vi "HFRR ADV v037.vi"() -> ()   [LabVIEW 2025] (continued)
                            n2633 = local write "Batch Ref Num :"(w3119) -> ()
                            n2634 = local write "FILE"(w3119) -> ()
                            n2635 = local write "EVENT LOG"(w3124) -> ()
                            n2636 = local write "TEST FILE NAM,E SAVED"(w3117) -> ()
                            n2637 = local write "Fuel Discription :"(w3119) -> ()
                            n2638 = local write "START TEMP"(w3117) -> ()
                            n2639 = local write "Remarks :"(w3119) -> ()
                            n2640 = local write "Main Dashboard Buttons"(T1."Imaging" ("Main Dashboard Buttons")) -> ()
                            n2641 = local write "Main Tab"(T2."Adv Scar" ("Main Tab")) -> ()
                            n2642 = property on="FRICVALZ 2" class="Bool (strict)"("DisabledEnum"=w3118) -> ()  [unwired: 2 in, 2 out]
                            n2643 = property on="FRICVALZ 3" class="Bool (strict)"("DisabledEnum"=w3118) -> ()  [unwired: 2 in, 2 out]
                            n2644 = property on="FRICVALZ 4" class="Bool (strict)"("DisabledEnum"=w3118) -> ()  [unwired: 2 in, 2 out]
                          }
                          frame #1 {
                            n2645 = Wait (ms)(milliseconds to wait=u32 1500) -> ()  [unwired: 1 out]
                          }
                          frame #2 {
                            n2646 = local write "Due Write"("VC;0") -> ()
                          }
                          frame #3 {
                            n2647 = Wait (ms)(milliseconds to wait=u32 1500) -> ()  [unwired: 1 out]
                          }
                          frame #4 {
                            n2648 = local write "Due Write"("VC;0") -> ()
                          }
                          frame #5 {
                            n2649 = Wait (ms)(milliseconds to wait=u32 1500) -> ()  [unwired: 1 out]
                          }
                          frame #6 {
                            n2650 = local write "Due Write"("ST;0") -> ()
                          }
                          frame #7 {
                            n2651 = local write "measured_stroke"(0.0 ("measured_stroke")) -> ()
                            n2652 = Wait (ms)(milliseconds to wait=u32 1500) -> ()  [unwired: 1 out]
                          }
                          frame #8 {
                            n2653 = local write "Due Write"("HE;0") -> ()
                            n2654 = local write "Humidity"(TRUE ("Humidity")) -> ()
                          }
                        }
                      }
                    }
                    n2655 = Divide(x=w3102, y=w3101) -> (x/y=w3105:dbl)
                    n2656 = Multiply(x=w3105, y=100.0) -> (x*y=w3103:dbl)
                    n2657 = local write "Test Duration Status"(w3103) -> ()
                  }
                }
              }
              frame #2 {
                n2658 = case shown="True" "Heater Button" {
                  tunnel: [0.0 ("output") w3240] -> w3218
                  frame False {
                    w3221 = TRUE ("tmpchk")
                    n2659 = local read "TEMP"() -> (w3222:dbl)
                    n2660 = local write "Temp ini"(w3222) -> ()
                    n2661 = local write "Reset 4"(w3221) -> ()
                    n2662 = local write "tmpchk"(w3221) -> ()
                    n2663 = local write "reinit"(TRUE ("reinit")) -> ()
                    n2664 = local write "manual temp log"(TRUE ("manual temp log")) -> ()
                  }
                  frame True {
                    # "Logic to turn off\nthe heater when \ntemp is not rising.\nTime - 60 sec\nDelta t- 5°c"
                    n2665 = local read "Temp ini"() -> (w3229:dbl)
                    n2666 = local read "Auto Start Test"() -> (w3225:bool)
                    n2667 = Less?(x=w3229, y=53.0) -> (x < y?=w3227:bool)
                    n2668 = case shown="False" w3225 {
                      frame False {
                        n2669 = local read "Set Temp"() -> (w3249:dbl)
                        n2670 = local read "TEMP"() -> (w3248:dbl)
                        n2671 = Subtract(x=w3249, y=w3248) -> (x-y=w3247:dbl)
                        n2672 = Absolute Value(x=w3247) -> (abs(x)=w3246:dbl)
                        n2673 = Less?(x=w3246, y=0.5) -> (x < y?=w3244:bool)
                        n2674 = case shown="True" w3244 {
                          tunnel: "manual temp log" -> [_ w3250]
                          frame False {
                          }
                          frame True {
                            n2675 = case shown="True" w3250 {
                              selector: w3250 -> [_ w3251]
                              frame False {
                              }
                              frame True {
                                # "#Event log"
                                n2676 = Not(x=w3251) -> (.not. x?=w3252:bool)
                                n2677 = local write "manual temp log"(w3252) -> ()
                                n2678 = local read "EVENT LOG"() -> (w3255:string)
                                n2679 = call "Event Log.vi"("Content"="Target Temperature reached", "EVENT LOG"=w3255) -> ("EVENT LOG"=w3254:string)  [unwired: 8 in, 1 out]
                                n2680 = local write "EVENT LOG"(w3254) -> ()
                              }
                            }
                          }
                        }
                      }
                      frame True {
                        n2681 = local write "manual temp log"(TRUE ("manual temp log")) -> ()
                      }
                    }
                    n2682 = And(x="tmpchk", y=w3227) -> (x .and. y?=w3230:bool)
                    n2683 = case shown="True" w3230 {
                      frame False {
                      }
                      frame True {
                        n2684 = call "Elapsed Time8"("Time Target (s)"=300.0, "Reset"="Reset 4") -> ("Time has Elapsed"=w3257:bool)  [unwired: 10 in, 7 out]
                        n2685 = flat-sequence {
                          tunnel: w3257 -> [_]
                          frame #0 {
                            n2686 = local write "Reset 4"(FALSE ("Reset 4")) -> ()
                          }
                        }
                        n2687 = case shown="True" w3257 {
                          frame False {
                          }
                          frame True {
                            n2688 = local read "Temp ini"() -> (w3264:dbl)
                            n2689 = Add(x=w3264, y=5.0) -> (x+y=w3262:dbl)
                            n2690 = local read "TEMP"() -> (w3265:dbl)
                            n2691 = Greater?(x=w3265, y=w3262) -> (0:w3263:bool)
                            n2692 = case shown="False" w3263 {
                              frame False {
                                n2693 = local write "Heater Button"(FALSE ("Heater Button")) -> ()
                              }
                              frame True {
                                n2694 = local write "tmpchk"(FALSE ("tmpchk")) -> ()
                              }
                            }
                          }
                        }
                      }
                    }
                    n2695 = local read "Set Temp"() -> (w3238:dbl)
                    n2696 = local read "TEMP"() -> (w3232:dbl)
                    n2697 = call-poly <vilib>:"PID.vi"("reinitialize? (F)"="reinit", "dt (s)"=-1.0, "process variable"=w3232, "setpoint"=w3238) -> ("output"=w3235:dbl)  [unwired: 6 in, 1 out]
                    n2698 = Subtract(x=w3238, y=w3232) -> (x-y=w3239:dbl)
                    n2699 = Add(x=w3238, y=0.5) -> (x+y=w3236:dbl)
                    n2700 = Greater Or Equal?(x=w3232, y=w3236) -> ()  [unwired: 1 out]
                    n2701 = Select(t=0.0, s=FALSE, f=w3235) -> (s? t:f=w3234:dbl)
                    "PID output" <- w3234
                    n2702 = flat-sequence {
                      tunnel: w3234 -> [w3268]
                      tunnel: [w3268] -> w3240
                      frame #0 {
                        n2703 = local write "reinit"(FALSE ("reinit")) -> ()
                      }
                    }
                    n2704 = Bundle(w3239, "output"=w3234, "TEMP"=w3232) -> ()  [unwired: 1 in, 1 out]
                  }
                }
                "PID-out" <- w3218
              }
              frame #3 {
                n2705 = local read "TEMP"() -> (w3270:dbl)
                n2706 = Greater Or Equal?(x=w3270, y="Set Temp 2") -> (x >= y?=w3275:bool)
                n2707 = case shown="True" w3275 {
                  tunnel: [FALSE TRUE] -> w3273
                  frame False {
                  }
                  frame True {
                  }
                }
                "Status 13" <- w3273
                n2708 = And(x=w3273, y="trip1 8") -> (x .and. y?=w3272:bool)
                n2709 = case shown="True" w3272 {
                  frame False {
                    n2710 = local write "Heater Trip Temp"(TRUE ("Heater Trip Temp")) -> ()
                  }
                  frame True {
                    w3278 = FALSE ("OK Button 2")
                    n2711 = case shown="True" "Heater Trip Temp" {
                      selector: "Heater Trip Temp" -> [_ w3280]
                      frame False {
                      }
                      frame True {
                        n2712 = Not(x=w3280) -> (.not. x?=w3279:bool)
                        n2713 = local read "EVENT LOG"() -> (w3283:string)
                        n2714 = local write "Heater Trip Temp"(w3279) -> ()
                        n2715 = call "Event Log.vi"("Content"="Heater Trip", "EVENT LOG"=w3283) -> ("EVENT LOG"=w3282:string)  [unwired: 8 in, 1 out]
                        n2716 = local write "EVENT LOG"(w3282) -> ()
                      }
                    }
                    n2717 = local write "RUN"(w3278) -> ()
                    n2718 = property on="Auto Start Test" class="Bool (strict)"("Value"=w3278) -> ()  [unwired: 2 in, 2 out]
                    n2719 = local write "Heater Button"(w3278) -> ()
                  }
                }
              }
            }
            n2720 = case shown="False" w2989 {
              frame False {
                n2721 = disable-structure shown="Disabled" {
                  frame Disabled {
                    n2722 = stacked-sequence {
                      frame #0 {
                        n2723 = local write "RUN"(FALSE ("OK Button 2")) -> ()
                      }
                      frame #1 {
                      }
                    }
                  }
                  frame Enabled {
                  }
                }
              }
              frame True {
              }
            }
          }
        }
        n2724 = local read "Reset Graph"() -> (w2886:bool)
        n2725 = case shown="True" w2886 {
          selector: w2886 -> [_ w2903]
          frame False {
          }
          frame True {
            w2917 = 0.0 ("X Scale.Range:Maximum")
            n2726 = Not(x=w2903) -> (.not. x?=w2902:bool)
            n2727 = local write "Reset Graph"(w2902) -> ()
            n2728 = property on="Electrical Contact Resistance ( % )" class="WFChart (strict)"("XScale.Maximum"=600.0 ("X Scale.Range:Maximum"), "XScale.Minimum"=0.0 ("X Scale.Range:Minimum"), "YScale.Maximum"=100.0 ("Y Scale.Range:Maximum"), "YScale.Minimum"=0.0 ("Y Scale.Range:Minimum")) -> ()  [unwired: 2 in, 2 out]
            n2729 = property on="Frictional Force ( N )" class="WFChart (strict)"("XScale.Maximum"=600.0 ("X Scale.Range:Maximum"), "XScale.Minimum"=0.0 ("X Scale.Range:Minimum"), "YScale.Maximum"=100.0 ("Y Scale.Range:Maximum"), "YScale.Minimum"=0.0 ("Y Scale.Range:Minimum")) -> ()  [unwired: 2 in, 2 out]
            n2730 = property on="Temperature ( Deg C )" class="WFChart (strict)"("XScale.Maximum"=600.0 ("X Scale.Range:Maximum"), "XScale.Minimum"=0.0 ("X Scale.Range:Minimum"), "YScale.Maximum"=100.0 ("Y Scale.Range:Maximum"), "YScale.Minimum"=0.0 ("Y Scale.Range:Minimum")) -> ()  [unwired: 2 in, 2 out]
            n2731 = property on="Stroke ( mm )" class="WFChart (strict)"("XScale.Maximum"=600.0 ("X Scale.Range:Maximum"), "XScale.Minimum"=0.0 ("X Scale.Range:Minimum"), "YScale.Maximum"=100.0 ("Y Scale.Range:Maximum"), "YScale.Minimum"=0.0 ("Y Scale.Range:Minimum")) -> ()  [unwired: 2 in, 2 out]
            n2732 = property on="Coefficient of Friction" class="WFChart (strict)"("XScale.Maximum"=600.0 ("X Scale.Range:Maximum"), "XScale.Minimum"=0.0 ("X Scale.Range:Minimum"), "YScale.Maximum"=100.0 ("Y Scale.Range:Maximum"), "YScale.Minimum"=0.0 ("Y Scale.Range:Minimum")) -> ()  [unwired: 2 in, 2 out]
            n2733 = property on="Electrical Contact Resistance ( % )" class="WFChart (strict)"("XScale.Minimum"=0.0 ("X Scale.Range:Minimum"), "XScale.Maximum"=600.0 ("X Scale.Range:Maximum"), "YScale.Minimum"=0.0 ("Y Scale.Range:Minimum"), "YScale.Maximum"=100.0 ("Y Scale.Range:Maximum")) -> ()  [unwired: 2 in, 2 out]
            n2734 = property on="Temperature ( Deg C )" class="WFChart (strict)"("XScale.Minimum"=0.0 ("X Scale.Range:Minimum"), "XScale.Maximum"=600.0 ("X Scale.Range:Maximum"), "YScale.Minimum"=0.0 ("Y Scale.Range:Minimum"), "YScale.Maximum"=100.0 ("Y Scale.Range:Maximum")) -> ()  [unwired: 2 in, 2 out]
            n2735 = property on="Coefficient of Friction" class="WFChart (strict)"("XScale.Minimum"=0.0 ("X Scale.Range:Minimum"), "XScale.Maximum"=600.0 ("X Scale.Range:Maximum"), "YScale.Maximum"=1.0 ("X Scale.Range:Minimum"), "YScale.Minimum"=0.0 ("X Scale.Range:Minimum")) -> ()  [unwired: 2 in, 2 out]
            n2736 = property on="Frictional Force ( N )" class="WFChart (strict)"("XScale.Maximum"=600.0 ("X Scale.Range:Maximum"), "XScale.Minimum"=w2917, "YScale.Maximum"=10.0 ("Y Scale.Range:Maximum"), "YScale.Minimum"=w2917) -> ()  [unwired: 2 in, 2 out]
            n2737 = property on="Stroke ( mm )" class="WFChart (strict)"("XScale.Maximum"=600.0 ("X Scale.Range:Maximum"), "XScale.Minimum"=0.0 ("X Scale.Range:Minimum"), "YScale.Maximum"=100.0 ("Y Scale.Range:Maximum"), "YScale.Minimum"=0.0 ("Y Scale.Range:Minimum")) -> ()  [unwired: 2 in, 2 out]
          }
        }
      }
      frame "Compare Files" {
        # "Elapsed time\ncof\nstroke\nAir temp\nTemp\nHumidity"
        n2738 = case shown="True" "RSTV1 2" {
          frame False {
          }
          frame True {
            n2739 = property on="Humidity ( %RH )" class="XYGraph (strict)"("Y Scale.Display Format:Precision"=u8 0 ("Y Scale.Format & Precision:Precision")) -> ()  [unwired: 2 in, 2 out]
            n2740 = property on="Humidity ( %RH )" class="XYGraph (strict)"("X Scale.Range:Minimum"=0.0, "X Scale.Range:Maximum"=75.0, "Y Scale.Range:Minimum"=48.0, "Y Scale.Range:Maximum"=58.0) -> ()  [unwired: 2 in, 2 out]
          }
        }
        n2741 = case shown="True" "RST CP 2" {
          frame False {
          }
          frame True {
            n2742 = property on="XY Graph 13" class="XYGraph (strict)"("Y Scale.Display Format:Precision"=u8 0 ("Y Scale.Format & Precision:Precision")) -> ()  [unwired: 2 in, 2 out]
            n2743 = property on="XY Graph 13" class="XYGraph (strict)"("X Scale.Range:Minimum"=0.0, "X Scale.Range:Maximum"=75.0, "Y Scale.Range:Minimum"=0.0, "Y Scale.Range:Maximum"=100.0) -> ()  [unwired: 2 in, 2 out]
          }
        }
        n2744 = case shown="True" "RST CP" {
          frame False {
          }
          frame True {
            n2745 = property on="Sample Temperature ( °C )" class="XYGraph (strict)"("Y Scale.Display Format:Precision"=u8 2 ("Y Scale.Format & Precision:Precision")) -> ()  [unwired: 2 in, 2 out]
            n2746 = property on="Sample Temperature ( °C )" class="XYGraph (strict)"("X Scale.Range:Minimum"=0.0, "X Scale.Range:Maximum"=75.0, "Y Scale.Range:Minimum"=58.0, "Y Scale.Range:Maximum"=62.0) -> ()  [unwired: 2 in, 2 out]
          }
        }
        n2747 = case shown="True" "RSTV1 3" {
          frame False {
          }
          frame True {
            n2748 = property on="Air Temperature  ( °C )" class="XYGraph (strict)"("Y Scale.Display Format:Precision"=u8 2 ("Y Scale.Format & Precision:Precision")) -> ()  [unwired: 2 in, 2 out]
            n2749 = property on="Air Temperature  ( °C )" class="XYGraph (strict)"("X Scale.Range:Minimum"=0.0 ("Y Scale.Range:Minimum"), "X Scale.Range:Maximum"=75.0 ("Y Scale.Range:Maximum"), "Y Scale.Range:Minimum"=20.0 ("X Scale.Range:Minimum"), "Y Scale.Range:Maximum"=26.0 ("X Scale.Range:Maximum")) -> ()  [unwired: 2 in, 2 out]
          }
        }
        n2750 = case shown="True" "RSTV1 4" {
          frame False {
          }
          frame True {
            n2751 = property on="Stroke ( mm )" class="XYGraph (strict)"("Y Scale.Display Format:Precision"=u8 2 ("Y Scale.Format & Precision:Precision")) -> ()  [unwired: 2 in, 2 out]
            n2752 = property on="Stroke ( mm )" class="XYGraph (strict)"("X Scale.Range:Minimum"=0.0 ("Y Scale.Range:Maximum"), "X Scale.Range:Maximum"=75.0 ("X Scale.Range:Minimum"), "Y Scale.Range:Minimum"=0.98, "Y Scale.Range:Maximum"=1.02) -> ()  [unwired: 2 in, 2 out]
          }
        }
        n2753 = case shown="True" "rstv2" {
          frame False {
          }
          frame True {
            n2754 = property on="Coefficient Of Friction" class="XYGraph (strict)"("Y Scale.Display Format:Precision"=u8 3 ("Y Scale.Format & Precision:Precision")) -> ()  [unwired: 2 in, 2 out]
            n2755 = property on="Coefficient Of Friction" class="XYGraph (strict)"("X Scale.Range:Minimum"=0.0 ("Y Scale.Range:Maximum"), "X Scale.Range:Maximum"=75.0, "Y Scale.Range:Minimum"=0.0, "Y Scale.Range:Maximum"=1.0 ("X Scale.Range:Minimum")) -> ()  [unwired: 2 in, 2 out]
          }
        }
        n2756 = case shown="True" "RST CP 3" {
          frame False {
          }
          frame True {
            n2757 = property on="Air Temp ( °C ) vs Humidity ( % RH )" class="XYGraph (strict)"("X Scale.Range:Minimum"=18.0, "X Scale.Range:Maximum"=28.0 ("X Scale.Range:Minimum"), "Y Scale.Range:Minimum"=30.0 ("X Scale.Range:Minimum"), "Y Scale.Range:Maximum"=70.0 ("X Scale.Range:Minimum")) -> ()  [unwired: 2 in, 2 out]
          }
        }
        n2758 = case shown="True" "OPEN 1" {
          frame False {
          }
          frame True {
            (unwired) 0  # existing file
            w3559 = "Choose a datalog file to open"  # prompt
            n2759 = local write "OPEN 1"(FALSE ("OPEN 1")) -> ()
            n2760 = String To Path(string="C:\\LAB-IQ\\Data\\") -> (path=w3544:path)
            n2761 = File Dialog(6:"*.dgf" ("pattern"), 7:w3559, 11:w3544) -> (0:w3542:errorcluster, 3:w3550:path)  [unwired: 4 in, 2 out]
            n2762 = Unbundle(w3542) -> ()  [unwired: 3 out]
            n2763 = Strip Path(path=w3550) -> (name=w3549:string)  [unwired: 1 out]
            n2764 = Path To String(path=w3550) -> (string=w3545:string)
            "string1" <- w3545
            n2765 = Match Pattern(string=w3549, regular expression=".dgf") -> (before substring=→"String Control":string)  [unwired: 1 in, 3 out]
            n2766 = Match Pattern(string=w3545, regular expression=".dgf" ("substring (\"\")")) -> (before substring=w3555:string)  [unwired: 1 in, 3 out]
            n2767 = Concatenate Strings(w3555, ".duf" ("Substring")) -> (w3551:string)
            n2768 = String To Path(string=w3551) -> (path=w3556:path)
            n2769 = call <vilib>:"Read Characters From File.vi"("file path (dialog if empty)"=w3556, "start of read offset (chars.:0)"=60 ("start of read offset (chars.: 0)")) -> ("character string"=→"String Control 2":string)  [unwired: 4 in, 3 out]
          }
        }
        n2770 = case shown="True" "OPEN 2" {
          frame False {
          }
          frame True {
            (unwired) 0  # existing file
            w3577 = "Choose a datalog file to open"  # prompt
            n2771 = local write "OPEN 2"(FALSE ("OPEN 1")) -> ()
            n2772 = String To Path(string="C:\\LAB-IQ\\Data\\") -> (path=w3562:path)
            n2773 = File Dialog(6:"*.dgf" ("pattern"), 7:w3577, 11:w3562) -> (0:w3560:errorcluster, 3:w3568:path)  [unwired: 4 in, 2 out]
            n2774 = Unbundle(w3560) -> ()  [unwired: 3 out]
            n2775 = Strip Path(path=w3568) -> (name=w3566:string)  [unwired: 1 out]
            n2776 = Path To String(path=w3568) -> (string=w3563:string)
            "string1 2" <- w3563
            n2777 = Match Pattern(string=w3566, regular expression=".dgf") -> (before substring=→"String Control 3":string)  [unwired: 1 in, 3 out]
            n2778 = Match Pattern(string=w3563, regular expression=".dgf" ("substring (\"\")")) -> (before substring=w3574:string)  [unwired: 1 in, 3 out]
            n2779 = Concatenate Strings(w3574, ".duf" ("Substring")) -> (w3571:string)
            n2780 = String To Path(string=w3571) -> (path=w3569:path)
            n2781 = call <vilib>:"Read Characters From File.vi"("file path (dialog if empty)"=w3569, "start of read offset (chars.:0)"=60 ("start of read offset (chars.: 0)")) -> ("character string"=→"String Control 4":string)  [unwired: 4 in, 3 out]
          }
        }
        n2782 = case shown="True" "OPEN 3" {
          frame False {
          }
          frame True {
            (unwired) 0  # existing file
            w3595 = "Choose a datalog file to open"  # prompt
            n2783 = local write "OPEN 3"(FALSE ("OPEN 1")) -> ()
            n2784 = String To Path(string="C:\\LAB-IQ\\Data\\") -> (path=w3580:path)
            n2785 = File Dialog(6:"*.dgf" ("pattern"), 7:w3595, 11:w3580) -> (0:w3578:errorcluster, 3:w3586:path)  [unwired: 4 in, 2 out]
            n2786 = Unbundle(w3578) -> ()  [unwired: 3 out]
            n2787 = Strip Path(path=w3586) -> (name=w3584:string)  [unwired: 1 out]
            n2788 = Path To String(path=w3586) -> (string=w3581:string)
            "string1 3" <- w3581
            n2789 = Match Pattern(string=w3584, regular expression=".dgf") -> (before substring=→"String Control 5":string)  [unwired: 1 in, 3 out]
            n2790 = Match Pattern(string=w3581, regular expression=".dgf" ("substring (\"\")")) -> (before substring=w3591:string)  [unwired: 1 in, 3 out]
            n2791 = Concatenate Strings(w3591, ".duf" ("Substring")) -> (w3588:string)
            n2792 = String To Path(string=w3588) -> (path=w3592:path)
            n2793 = call <vilib>:"Read Characters From File.vi"("file path (dialog if empty)"=w3592, "start of read offset (chars.:0)"=60 ("start of read offset (chars.: 0)")) -> ("character string"=→"String Control 6":string)  [unwired: 4 in, 3 out]
          }
        }
        n2794 = case shown="True" "OPEN 4" {
          frame False {
          }
          frame True {
            (unwired) 0  # existing file
            w3613 = "Choose a datalog file to open"  # prompt
            n2795 = local write "OPEN 4"(FALSE ("OPEN 1")) -> ()
            n2796 = String To Path(string="C:\\LAB-IQ\\Data\\") -> (path=w3598:path)
            n2797 = File Dialog(6:"*.dgf" ("pattern"), 7:w3613, 11:w3598) -> (0:w3596:errorcluster, 3:w3604:path)  [unwired: 4 in, 2 out]
            n2798 = Unbundle(w3596) -> ()  [unwired: 3 out]
            n2799 = Strip Path(path=w3604) -> (name=w3602:string)  [unwired: 1 out]
            n2800 = Path To String(path=w3604) -> (string=w3599:string)
            "string1 4" <- w3599
            n2801 = Match Pattern(string=w3602, regular expression=".dgf") -> (before substring=→"String Control 7":string)  [unwired: 1 in, 3 out]
            n2802 = Match Pattern(string=w3599, regular expression=".dgf" ("substring (\"\")")) -> (before substring=w3609:string)  [unwired: 1 in, 3 out]
            n2803 = Concatenate Strings(w3609, ".duf" ("Substring")) -> (w3606:string)
            n2804 = String To Path(string=w3606) -> (path=w3610:path)
            n2805 = call <vilib>:"Read Characters From File.vi"("file path (dialog if empty)"=w3610, "start of read offset (chars.:0)"=60 ("start of read offset (chars.: 0)")) -> ("character string"=→"String Control 8":string)  [unwired: 4 in, 3 out]
          }
        }
      }
      frame "About" {
        # "Elapsed time\ncof\nstroke\nmean pos\nTemp\nHumidity"
        n2806 = disable-structure shown="Disabled" {
          frame Disabled {
            n2807 = case shown="True" "Export" {
              frame False {
              }
              frame True {
                w3635 = "                                      " ("string")
                w3637 = "\r"
                (unwired) i16 6 ("width (-)")
                w3714 = "\r"
                w3646 = "\r"
                n2808 = local write "Export"(FALSE ("Export")) -> ()
                n2809 = local read "String 29"() -> (w3683:string)
                n2810 = local read "String 34"() -> (w3671:string)
                n2811 = local read "String 35"() -> (w3666:string)
                n2812 = local read "String 37"() -> (w3662:string)
                n2813 = local read "String 36"() -> (w3659:string)
                n2814 = local read "String 38"() -> (w3656:string)
                n2815 = local read "String 39"() -> (w3653:string)
                n2816 = Match Pattern(string=w3683, regular expression=".dwm") -> (before substring=w3679:string)  [unwired: 1 in, 3 out]
                "before substring" <- w3679
                n2817 = local read "S 38"() -> (w3674:string)
                n2818 = local read "S 39"() -> (w3667:string)
                n2819 = local read "Temperature before test 2"() -> (w3703:dbl)
                n2820 = local read "Temperature after test 2"() -> (w3708:dbl)
                n2821 = local read "Humidity before test 2"() -> (w3689:dbl)
                n2822 = local read "Humidity after test 2"() -> (w3704:dbl)
                n2823 = local read "MWSD 2"() -> (w3700:dbl)
                n2824 = local read "WS1.4 2"() -> (w3716:dbl)
                n2825 = local read "HCF 2"() -> (w3712:dbl)
                n2826 = local read "AVP 2"() -> (w3701:dbl)
                n2827 = Concatenate Strings("1," ("string"), w3674) -> (w3673:string)
                n2828 = Concatenate Strings("2," ("string"), w3671) -> (w3670:string)
                n2829 = Concatenate Strings("3," ("string"), w3667) -> (w3669:string)
                n2830 = Concatenate Strings("4," ("string"), w3666) -> (w3665:string)
                n2831 = Concatenate Strings("5," ("string"), w3662) -> (w3663:string)
                n2832 = Concatenate Strings("6," ("string"), w3659) -> (w3660:string)
                n2833 = Concatenate Strings("7," ("string"), w3656) -> (w3657:string)
                n2834 = Concatenate Strings("8," ("string"), w3653) -> (w3654:string)
                n2835 = local read "Sample ID"() -> (w3721:string)
                n2836 = case shown="\"xlx\"" "Select File Type" {
                  tunnel: w3679 -> [w3724 w3726 w3728]
                  tunnel: [w3722 w3727 w3729] -> w3678
                  frame "xlx" {
                    n2837 = Concatenate Strings(w3724, ".xls" ("string")) -> (w3722:string)
                  }
                  frame "csv" {
                    n2838 = Concatenate Strings(w3726, ".csv" ("string")) -> (w3727:string)
                  }
                  frame "txt" {
                    n2839 = Concatenate Strings(w3728, ".txt" ("string")) -> (w3729:string)
                  }
                }
                n2840 = local read "Test Date"() -> (w3720:string)
                n2841 = local read "String 45"() -> (w3634:string)
                n2842 = local read "String 31"() -> (w3719:string)
                n2843 = local read "String 32"() -> (w3718:string)
                n2844 = local read "TITTLE"() -> (w3642:string)
                n2845 = Number To Fractional String(number=w3689, width (-)=i16 6, precision (6)=i16 2) -> (F-format string=w3688:string)  [unwired: 1 in]
                n2846 = Number To Fractional String(number=w3703, width (-)=i16 6, precision (6)=i16 2) -> (F-format string=w3709:string)  [unwired: 1 in]
                n2847 = Number To Fractional String(number=w3704, width (-)=i16 6, precision (6)=i16 2) -> (F-format string=w3702:string)  [unwired: 1 in]
                n2848 = Number To Fractional String(number=w3708, width (-)=i16 6, precision (6)=i16 2) -> (F-format string=w3707:string)  [unwired: 1 in]
                n2849 = Number To Fractional String(number=w3700, width (-)=i16 6, precision (6)=i16 2) -> (F-format string=w3698:string)  [unwired: 1 in]
                n2850 = Number To Fractional String(number=w3701, width (-)=i16 6, precision (6)=i16 2) -> (F-format string=w3699:string)  [unwired: 1 in]
                n2851 = Number To Fractional String(number=w3712, width (-)=i16 6, precision (6)=i16 2) -> (F-format string=w3713:string)  [unwired: 1 in]
                n2852 = Number To Fractional String(number=w3716, precision (6)=i16 2) -> (F-format string=w3717:string)  [unwired: 2 in]
                n2853 = local read "s.NO"() -> (w3636:string)
                n2854 = Concatenate Strings("=" ("string"), w3642) -> (w3641:string)
                n2855 = Concatenate Strings("S.No," ("string"), "                                       Parameters" ("string")) -> (w3647:string)
                n2856 = Concatenate Strings(w3714, w3673, w3688, w3714, w3670, w3709, w3714, w3669, w3702, w3714, w3665, w3707, w3714, w3663, w3698, w3714, w3660, w3699, w3714, w3657, w3713, w3714, w3654, w3717) -> (w3676:string)
                n2857 = Concatenate Strings(w3646, "," ("string"), w3634, w3636, w3635, w3718, w3721, w3635, w3719, w3720, w3646) -> (w3644:string)
                n2858 = local read "Tested by"() -> (w3650:string)
                n2859 = local read "String 33"() -> (w3651:string)
                n2860 = Concatenate Strings("," ("string"), "                                                                             " ("string")) -> (w3639:string)
                n2861 = Concatenate Strings(w3641, w3637, w3644, w3637, w3647, w3676, w3637, w3639, w3651, w3650) -> (→"export":string)
                n2862 = String To Path(string=w3678) -> (path=w3685:path)
                n2863 = local read "export"() -> (w3680:string)
                n2864 = call <vilib>:"Write Characters To File.vi"("append to file? (new file:F)"=FALSE, "character string"=w3680, "file path (dialog if empty)"=w3685) -> ()  [unwired: 2 in, 1 out]
              }
            }
          }
          frame Enabled {
          }
        }
        n2865 = case shown="True" "OK Button 17" {
          frame False {
          }
          frame True {
            (unwired) 0  # existing file
            w3938 = "Choose a datalog file to open"  # prompt
            n2866 = local write "OK Button 17"(FALSE ("OK Button 17")) -> ()
            n2867 = local read "String"() -> (w3933:string)
            n2868 = String To Path(string=w3933) -> (path=w3934:path)
            n2869 = File Dialog(6:"*.duf" ("pattern"), 7:w3938, 11:w3934) -> (0:w3925:errorcluster, 3:w3944:path)  [unwired: 4 in, 2 out]
            n2870 = Unbundle(w3925) -> ()  [unwired: 3 out]
            n2871 = Open/Create/Replace File "Open File"(file path (use dialog)=w3944) -> (refnum out=w3936:refnum<file>)  [unwired: 5 in, 2 out]
            n2872 = Strip Path(path=w3944) -> (name=w3942:string)  [unwired: 1 out]
            n2873 = Path To String(path=w3944) -> (string=w3927:string)
            n2874 = while {
              tunnel: w3936 -> [w3948]
              i -> [w3945]
              stop <- w3946 continue-if-true
              (unwired) TRUE ("line mode (F)")
              n2875 = Read from Text File "Read File"(file (use dialog)=w3948) -> (text=w3947:string)  [unwired: 3 in, 3 out]
              n2876 = local write "Numeric 16"(w3945) -> ()
              n2877 = String Length(string=w3947) -> (length=w3950:i32)
              n2878 = Greater?(x=w3950, y=1) -> (0:w3946:bool)
            }
            n2879 = local write "String 29"(w3927) -> ()
            n2880 = Search and Replace String(input string=w3927, search string=".duf", replace string=".dgf" ("replace string (\"\")")) -> (result string=→"String Indicator 4":string)  [unwired: 5 in, 3 out]
            n2881 = Match Pattern(string=w3942, regular expression=".dwm") -> (before substring=w3926:string)  [unwired: 1 in, 3 out]
            "String Indicator" <- w3926
            n2882 = Match Pattern(string=w3927, regular expression=".dwm" ("substring (\"\")")) -> (before substring=w3928:string)  [unwired: 1 in, 3 out]
            "String Indicator 3" <- w3928
            n2883 = local write "TITTLE 2"(w3926) -> ()
            n2884 = String To Path(string=w3928) -> (path=w3935:path)
            "path" <- w3935
            n2885 = call <vilib>:"Read Characters From File.vi"("file path (dialog if empty)"=w3935, "start of read offset (chars.:0)"=60 ("start of read offset (chars.: 0)")) -> ("character string"=→"String Indicator 2":string)  [unwired: 4 in, 3 out]
          }
        }
        n2886 = call <vilib>:"Query Available Printers.vi"() -> ("system configured printers"=w3627:string[])  [unwired: 9 in, 2 out]
        "System Configured Printers 2" <- w3627
        n2887 = local read "OK Button 16"() -> (w3624:bool)
        n2888 = case shown="True" "OK Button 16" {
          frame False {
          }
          frame True {
            n2889 = stacked-sequence {
              frame #0 {
                n2890 = local read "Numeric 16"() -> (w3952:i32)
                n2891 = local write "Numeric 10"(w3952) -> ()
              }
              frame #1 {
                n2892 = local read "String 29"() -> (w3955:string)
                n2893 = String To Path(string=w3955) -> (path=w3954:path)
                n2894 = Open/Create/Replace File "Open File"(file path (use dialog)=w3954) -> (refnum out=w3956:refnum<file>)  [unwired: 5 in, 2 out]
                n2895 = for {
                  N: 16 -> [_]
                  tunnel: w3956 -> [w3963]
                  i -> [w3959]
                  (unwired) TRUE ("line mode (F)")
                  n2896 = Read from Text File "Read File"(file (use dialog)=w3963) -> (text=w3957:string)  [unwired: 3 in, 3 out]
                  n2897 = Match Pattern(string=w3957, regular expression="(") -> (after substring=w3962:string)  [unwired: 1 in, 3 out]
                  n2898 = Match Pattern(string=w3962, regular expression=")") -> (before substring=w3958:string)  [unwired: 1 in, 3 out]
                  n2899 = case shown="1" w3959 {
                    tunnel: w3958 -> [w3964 w3965 _ _ w3966 w3967 w3968 w3970 w3972 w3974 w3976 w3978 w3980 w3982 _]
                    tunnel: w3957 -> [_ _ _ _ _ _ _ _ _ _ _ _ _ _ _]
                    frame 0 {
                      "TITTLE" <- w3964
                    }
                    frame 1 {
                      "Sample ID" <- w3965
                    }
                    frame 2 {
                    }
                    frame 3 {
                    }
                    frame 4 {
                      "Test Date" <- w3966
                    }
                    frame 5 {
                      "Tested by" <- w3967
                    }
                    frame 6 {
                      n2900 = Fract/Exp String To Number(string=w3968) -> (number=→"Humidity before test 2":dbl)  [unwired: 3 in, 1 out]
                    }
                    frame 7 {
                      n2901 = Fract/Exp String To Number(string=w3970) -> (number=→"Temperature before test 2":dbl)  [unwired: 3 in, 1 out]
                    }
                    frame 8 {
                      n2902 = Fract/Exp String To Number(string=w3972) -> (number=→"Humidity after test 2":dbl)  [unwired: 3 in, 1 out]
                    }
                    frame 9 {
                      n2903 = Fract/Exp String To Number(string=w3974) -> (number=→"Temperature after test 2":dbl)  [unwired: 3 in, 1 out]
                    }
                    frame 10 {
                      n2904 = Fract/Exp String To Number(string=w3976) -> (number=→"MWSD 2":dbl)  [unwired: 3 in, 1 out]
                    }
                    frame 11 {
                      n2905 = Fract/Exp String To Number(string=w3978) -> (number=→"AVP 2":dbl)  [unwired: 3 in, 1 out]
                    }
                    frame 12 {
                      n2906 = Fract/Exp String To Number(string=w3980) -> (number=→"HCF 2":dbl)  [unwired: 3 in, 1 out]
                    }
                    frame 13 {
                      n2907 = Fract/Exp String To Number(string=w3982) -> (number=→"WS1.4 2":dbl)  [unwired: 3 in, 1 out]
                    }
                    frame 14, Default {
                    }
                  }
                }
              }
              frame #2 {
              }
            }
            n2908 = local write "OK Button 16"(FALSE ("OK Button 13")) -> ()
          }
        }
        n2909 = Index Array(array=w3627, index="Select Printer 3") -> (element=w3629:string)
        "Selected Printer" <- w3629
        n2910 = case shown="True" w3624 {
          frame False {
          }
          frame True {
            n2911 = flat-sequence {
              frame #0 {
              }
              frame #1 {
                n2912 = Wait (ms)(milliseconds to wait=u32 100) -> ()  [unwired: 1 out]
              }
              frame #2 {
                n2913 = local write "OK Button 16"(FALSE ("Print 3")) -> ()
              }
            }
          }
        }
        n2914 = case shown="True" "Print" {
          tunnel: w3629 -> [_ w3921]
          frame False {
          }
          frame True {
            (unwired) i16 6 ("width (-)")
            (unwired) "TESTED BY : "
            (unwired) "TESTED DATE :"
            (unwired) "SAMPLE ID : "
            (unwired) "SAMPLE DESIGN : "
            w3879 = "\r"
            w3896 = "\r"
            # "add image"
            n2915 = local read "Sample ID"() -> (w3869:string)
            n2916 = local read "Tested by"() -> (w3872:string)
            n2917 = local read "String 34"() -> (w3859:string)
            n2918 = local read "String 45"() -> (w3839:string)
            n2919 = local read "String 35"() -> (w3854:string)
            n2920 = local read "String 37"() -> (w3852:string)
            n2921 = local read "String 32"() -> (w3874:string)
            n2922 = local read "String 36"() -> (w3849:string)
            n2923 = local read "String 31"() -> (w3873:string)
            n2924 = local read "Test Date"() -> (w3870:string)
            n2925 = local read "String 33"() -> (w3875:string)
            n2926 = local read "String 38"() -> (w3845:string)
            n2927 = local read "String 39"() -> (w3842:string)
            n2928 = local write "Print"(FALSE ("Print FF")) -> ()
            n2929 = local read "S 39"() -> (w3857:string)
            n2930 = local read "S 38"() -> (w3864:string)
            n2931 = local read "Temperature before test 2"() -> (w3895:dbl)
            n2932 = local read "Temperature after test 2"() -> (w3885:dbl)
            n2933 = local read "Humidity before test 2"() -> (w3910:dbl)
            n2934 = local read "Humidity after test 2"() -> (w3894:dbl)
            n2935 = local read "MWSD 2"() -> (w3899:dbl)
            n2936 = local read "WS1.4 2"() -> (w3877:dbl)
            n2937 = Concatenate Strings("2)" ("string"), w3859) -> (w3860:string)
            n2938 = Concatenate Strings("3)" ("string"), w3857) -> (w3858:string)
            n2939 = Concatenate Strings("1)" ("string"), w3864) -> (w3863:string)
            n2940 = Concatenate Strings("4)" ("string"), w3854) -> (w3855:string)
            n2941 = Concatenate Strings("5)" ("string"), w3852) -> (w3851:string)
            n2942 = Concatenate Strings("6)" ("string"), w3849) -> (w3848:string)
            n2943 = Concatenate Strings("7)" ("string"), w3845) -> (w3846:string)
            n2944 = Concatenate Strings("8)" ("string"), w3842) -> (w3843:string)
            n2945 = local read "HCF 2"() -> (w3881:dbl)
            n2946 = local read "AVP 2"() -> (w3898:dbl)
            n2947 = local read "s.NO"() -> (w3840:string)
            n2948 = call <vilib>:"New Report.vi"("report type"=enum16{"Standard Report", "HTML"}."Standard Report") -> ("report out"=w3919:refnum<class "NI_report.lvclass">, "error out"=w3918:errorcluster)  [unwired: 13 in]
            n2949 = local read "TITTLE"() -> (w3871:string)
            n2950 = Concatenate Strings(w3896, w3839, w3840, w3896, w3874, w3869, w3896, w3873, w3870, w3896, w3875, w3872, w3896) -> (w3889:string)
            "test by" <- w3889
            n2951 = Number To Fractional String(number=w3895, width (-)=i16 6, precision (6)=i16 2) -> (F-format string=w3884:string)  [unwired: 1 in]
            n2952 = Number To Fractional String(number=w3894, width (-)=i16 6, precision (6)=i16 2) -> (F-format string=w3897:string)  [unwired: 1 in]
            n2953 = Number To Fractional String(number=w3910, width (-)=i16 6, precision (6)=i16 2) -> (F-format string=w3915:string)  [unwired: 1 in]
            n2954 = Number To Fractional String(number=w3899, width (-)=i16 6, precision (6)=i16 2) -> (F-format string=w3901:string)  [unwired: 1 in]
            n2955 = Number To Fractional String(number=w3885, width (-)=i16 6, precision (6)=i16 2) -> (F-format string=w3886:string)  [unwired: 1 in]
            n2956 = Number To Fractional String(number=w3898, width (-)=i16 6, precision (6)=i16 2) -> (F-format string=w3900:string)  [unwired: 1 in]
            n2957 = Number To Fractional String(number=w3881, width (-)=i16 6, precision (6)=i16 2) -> (F-format string=w3880:string)  [unwired: 1 in]
            n2958 = Number To Fractional String(number=w3877, precision (6)=i16 2) -> (F-format string=w3876:string)  [unwired: 2 in]
            n2959 = call-dynamic "Set Report Header Text.vi"("report in"=w3919, "center header text"=w3871, "error in (no error)"=w3918) -> ("report out"=w3890:refnum<class "NI_report.lvclass">, "error out"=w3891:errorcluster)  [unwired: 11 in]
            n2960 = Concatenate Strings(w3879, w3863, w3915, w3879, w3860, w3884, w3879, w3858, w3897, w3879, w3855, w3886, w3879, w3851, w3901, w3879, w3848, w3900, w3879, w3846, w3880, w3879, w3843, w3876) -> (w3867:string)
            "export 2" <- w3867
            n2961 = call-poly <vilib>:"Append Report Text.vi"("report in"=w3890, "text"=w3889, "error in (no error)"=w3891) -> ("report out"=w3893:refnum<class "NI_report.lvclass">, "error out"=w3892:errorcluster)  [unwired: 9 in, 2 out]
            n2962 = local read "test by"() -> (w3866:string)
            n2963 = local read "TITTLE"() -> (w3868:string)
            n2964 = call-poly <vilib>:"Append Report Text.vi"("report in"=w3893, "error in (no error)"=w3892) -> ("report out"=w3914:refnum<class "NI_report.lvclass">, "error out"=w3912:errorcluster)  [unwired: 10 in, 2 out]
            n2965 = Concatenate Strings(w3868, w3867, w3866) -> (→"output":string)
            n2966 = call-poly <vilib>:"Append Report Text.vi"("report in"=w3914, "text"=w3867, "error in (no error)"=w3912) -> ("report out"=w3913:refnum<class "NI_report.lvclass">, "error out"=w3911:errorcluster)  [unwired: 9 in, 2 out]
            n2967 = call-dynamic "Print Report.vi"("report in"=w3913, "printer name (default)"=w3921, "error in (no error)"=w3911) -> ("report out"=w3923:refnum<class "NI_report.lvclass">, "error out"=w3924:errorcluster)  [unwired: 11 in]
            n2968 = call-dynamic "Dispose Report.vi"("report in"=w3923, "error in (no error)"=w3924) -> ()  [unwired: 13 in, 1 out]
          }
        }
        n2969 = case shown="True" "Print 2" {
          frame False {
          }
          frame True {
            n2970 = flat-sequence {
              frame #0 {
                n2971 = local read "s.NO"() -> (→"s.NO 2":string)
                n2972 = Wait (ms)(milliseconds to wait=u32 20) -> ()  [unwired: 1 out]
                n2973 = local read "Sample ID  3"() -> (→"Sample ID  6":string)
                n2974 = local read "Sample ID  4"() -> (→"Sample ID  7":string)
                n2975 = local read "Sample ID"() -> (→"Sample ID  2":string)
                n2976 = local read "Tested by"() -> (→"Tested by 2":string)
                n2977 = local read "Test Date"() -> (→"Test Date 2":string)
                n2978 = local read "Humidity after test 3"() -> (→"Humidity after test 4":dbl)
                n2979 = local read "Ref A Test Date :"() -> (→"TITTLE 4":string)
                n2980 = local read "Temperature before test 3"() -> (w3746:dbl)
                n2981 = local read "Temperature before test 3"() -> (→"Temperature after test 5":dbl)
                n2982 = local read "Temperature after test 3"() -> (→"Temperature after test 4":dbl)
                n2983 = local read "Humidity before test 3"() -> (→"Humidity before test 4":dbl)
                n2984 = local write "Temperature before test 3"(w3746) -> ()
                n2985 = local read "image data"() -> (w3737:T16)
                n2986 = String To Path(string="C:\\LAB-IQ\\im\\Temp_resized.jpg") -> (path=w3738:path)
                "path 2" <- w3738
                n2987 = call <vilib>:"Write JPEG File.vi"("image data"=w3737, "path to JPEG file"=w3738) -> ()  [unwired: 8 in, 2 out]
                "Ref A Test Date :" <- "Ref A Test Date :"
                "Ref B Test Date :" <- "Ref B Test Date :"
                "Ref B Scar Value :" <- "Ref B Scar Value :"
                "Ref A Scar Value :" <- "Ref A Scar Value :"
              }
              frame #1 {
                (unwired) HTML_Report_Image_Alignment."MIDDLE" ("alignment (default)")
                w3774 = u16 0 items=["portrait", "landscape"] ("orientation (portrait)")
                (unwired) HTML_Report_Image_Alignment."ABSMIDDLE" ("alignment (default)")
                (unwired) "TESTED BY : "
                (unwired) "TESTED DATE :"
                (unwired) "SAMPLE ID : "
                (unwired) "SAMPLE DESIGN : "
                w3807 = "\r"
                # "add image"
                n2988 = Wait (ms)(milliseconds to wait=u32 20) -> ()  [unwired: 1 out]
                n2989 = local read "Sample ID  2"() -> (w3800:string)
                n2990 = local read "Wear Scar X"() -> (w3772:dbl)
                "Length ( microns ) 2" <- w3772
                n2991 = local read "Wear Scar Y"() -> (w3771:dbl)
                "Wear Scar Y ( microns ) :" <- w3771
                n2992 = local read "Test Date 2"() -> (w3801:string)
                n2993 = local read "Tested by 2"() -> (w3802:string)
                n2994 = local read "String 46"() -> (w3798:string)
                n2995 = local read "String 48"() -> (w3804:string)
                n2996 = local read "String 47"() -> (w3803:string)
                n2997 = local read "String 49"() -> (w3805:string)
                n2998 = local read "String 10"() -> (w3758:string)
                n2999 = local read "s.NO 2"() -> (w3799:string)
                n3000 = Add(x=w3772, y=w3771) -> (x+y=w3770:dbl)
                n3001 = call <vilib>:"New Report.vi"("report type"=enum16{"Standard Report", "HTML"}."HTML") -> ("report out"=w3778:refnum<class "NI_report.lvclass">, "error out"=w3776:errorcluster)  [unwired: 13 in]
                n3002 = Concatenate Strings(w3807, w3798, w3799, w3807, w3804, w3800, w3807, w3803, w3801, w3807, w3805, w3802, w3807) -> (→"test by 2":string)
                n3003 = Concatenate Strings("C:\\LAB-IQ\\Data\\" ("string"), w3758, ".jpg" ("string")) -> ()  [unwired: 1 out]
                n3004 = Divide(x=w3770, y=2.0) -> (x/y=→"Mean Wear ( microns) :":dbl)
                n3005 = call-dynamic "Set Report Orientation.vi"("report in"=w3778, "orientation (portrait)"=w3774, "error in (no error)"=w3776) -> ("report out"=w3777:refnum<class "NI_report.lvclass">, "error out"=w3775:errorcluster)  [unwired: 11 in]
                n3006 = for {
                  N: 5 -> [_]
                  tunnel: w3777 -> [w3828]
                  tunnel: [w3827] -> w3756
                  tunnel: w3775 -> [w3826]
                  tunnel: [w3825] -> w3755
                  n3007 = call-dynamic "Set Report Tab Width.vi"("report in"=w3828, "error in (no error)"=w3826) -> ("report out"=w3827:refnum<class "NI_report.lvclass">, "error out"=w3825:errorcluster)  [unwired: 12 in]
                }
                n3008 = local read "TITTLE"() -> (w3773:string)
                n3009 = call-dynamic "Set Report Header Text.vi"("report in"=w3756, "center header text"=w3773, "error in (no error)"=w3755) -> ("report out"=w3794:refnum<class "NI_report.lvclass">, "error out"=w3793:errorcluster)  [unwired: 11 in]
                n3010 = for {
                  N: 1 -> [_]
                  tunnel: [w3832] -> w3780
                  tunnel: [w3831] -> w3779
                  tunnel: w3794 -> [w3830]
                  tunnel: w3793 -> [w3829]
                  n3011 = call-dynamic "New Report Line.vi"("report in"=w3830, "error in (no error)"=w3829) -> ("report out"=w3832:refnum<class "NI_report.lvclass">, "error out"=w3831:errorcluster)  [unwired: 12 in]
                }
                n3012 = for {
                  N: 2 -> [_]
                  tunnel: [w3824] -> w3786
                  tunnel: [w3823] -> w3785
                  tunnel: w3780 -> [w3822]
                  tunnel: w3779 -> [w3821]
                  n3013 = call-dynamic "New Report Line.vi"("report in"=w3822, "error in (no error)"=w3821) -> ("report out"=w3824:refnum<class "NI_report.lvclass">, "error out"=w3823:errorcluster)  [unwired: 12 in]
                }
                n3014 = for {
                  N: 25 -> [_]
                  tunnel: w3786 -> [w3820]
                  tunnel: w3785 -> [w3818]
                  tunnel: [w3819] -> w3789
                  tunnel: [w3817] -> w3788
                  n3015 = call-dynamic "Set Report Tab Width.vi"("report in"=w3820, "error in (no error)"=w3818) -> ("report out"=w3819:refnum<class "NI_report.lvclass">, "error out"=w3817:errorcluster)  [unwired: 12 in]
                }
                n3016 = control-ref of="Tab Control 9"() -> (w3784:refnum<vi>)
                n3017 = call-dynamic "Append Control Image to Report.vi"("report in"=w3789, "alignment (default)"=HTML_Report_Image_Alignment."ABSMIDDLE", "ctrl reference"=w3784, "error in (no error)"=w3788) -> ("report out"=w3783:refnum<class "NI_report.lvclass">, "error out"=w3782:errorcluster)  [unwired: 8 in, 2 out]
                n3018 = for {
                  N: 3 -> [_]
                  tunnel: [w3816] -> w3767
                  tunnel: [w3815] -> w3766
                  tunnel: w3783 -> [w3814]
                  tunnel: w3782 -> [w3813]
                  n3019 = call-dynamic "New Report Line.vi"("report in"=w3814, "error in (no error)"=w3813) -> ("report out"=w3816:refnum<class "NI_report.lvclass">, "error out"=w3815:errorcluster)  [unwired: 12 in]
                }
                n3020 = for {
                  N: 100 -> [_]
                  tunnel: w3767 -> [w3812]
                  tunnel: w3766 -> [w3810]
                  tunnel: [w3811] -> w3763
                  tunnel: [w3809] -> w3761
                  n3021 = call-dynamic "Set Report Tab Width.vi"("report in"=w3812, "error in (no error)"=w3810) -> ("report out"=w3811:refnum<class "NI_report.lvclass">, "error out"=w3809:errorcluster)  [unwired: 12 in]
                }
                n3022 = String To Path(string="C:\\LAB-IQ\\im\\Temp_resized.jpg") -> (path=w3753:path)
                n3023 = call-poly <vilib>:"Append Image to Report.vi"("report in"=w3763, "path or URL of image"=w3753, "error in (no error)"=w3761) -> ("report out"=w3762:refnum<class "NI_report.lvclass">, "error out"=w3760:errorcluster)  [unwired: 9 in, 2 out]
                n3024 = call-poly <vilib>:"Open HTML Report in Browser.vi"("report in"=w3762, "error in (no error)"=w3760) -> ("report out"=w3797:refnum<class "NI_report.lvclass">, "error out"=w3796:errorcluster)  [unwired: 11 in, 1 out]
                n3025 = call-dynamic "Dispose Report.vi"("report in"=w3797, "error in (no error)"=w3796) -> ()  [unwired: 13 in, 1 out]
              }
              frame #2 {
              }
              frame #3 {
                n3026 = disable-structure shown="Disabled" {
                  frame Disabled {
                    n3027 = local read "String 10"() -> (w3837:string)
                    n3028 = Concatenate Strings("C:\\LAB-IQ-NXT\\Data\\" ("string"), w3837, ".jpg" ("string")) -> (w3835:string)
                    n3029 = String To Path(string=w3835) -> (path=w3834:path)
                    n3030 = Delete(path (use dialog)=w3834) -> ()  [unwired: 4 in, 3 out]
                  }
                  frame Enabled {
                  }
                }
                n3031 = local write "Print 2"(FALSE ("Print")) -> ()
              }
            }
          }
        }
      }
    }
    n3032 = Wait (ms)(milliseconds to wait=u32 50) -> ()  [unwired: 1 out]
    n3033 = Wait (ms)(milliseconds to wait=u32 50) -> ()  [unwired: 1 out]
    n3034 = local read "Quit"() -> (w2179:bool)
  }
  n3035 = VISA Close(VISA resource name=w41, error in (no error)=w40) -> ()  [unwired: 1 out]
  n3036 = while {
    stop <- w3988 stop-if-true
    n3037 = local read "Auto Start Test"() -> (w3986:bool)
    n3038 = local read "RUN"() -> (w3985:bool)
    n3039 = Wait (ms)(milliseconds to wait=u32 1000) -> ()  [unwired: 1 out]
    n3040 = Or(x=w3985, y=w3986) -> (x .or. y?=w3984:bool)
    n3041 = case shown="True" w3984 {
      frame False {
      }
      frame True {
        n3042 = local read "LVDT STROKE Actual"() -> (w3989:dbl)
        n3043 = In Range and Coerce(upper limit=1.2, x=w3989, lower limit=0.6) -> (In Range?=w3992:bool)  [unwired: 1 out]
        n3044 = call-poly <vilib>:"Random Number (Range).vi"("lower bound (0)"=0.998 ("upper bound (100)"), "upper bound (100)"=1.003) -> ("number"=w3990:dbl)  [unwired: 9 in]
        n3045 = case shown="True" w3992 {
          tunnel: [w3997 w3998] -> w3991
          tunnel: w3990 -> [_ w3998]
          tunnel: w3989 -> [w3997 _]
          frame False {
          }
          frame True {
          }
        }
        "LVDT STROKE DISPLAY" <- w3991
      }
    }
    n3046 = local read "Quit"() -> (w3988:bool)
  }
  n3047 = while {
    tunnel: [w4015] -> w49
    shift-right: [w4008] -> _
    shift-left: 0.0 -> [w4011]
    shift-right: [w4007] -> _
    shift-left: 0.0 -> [w4010]
    shift-right: [w4006] -> _
    shift-left: 100.0 ("vc_cmd") -> [w4009]
    stop <- w4015 stop-if-true
    # "PID LOGIC"
    n3048 = local read "run test Calibration"() -> (w4003:bool)
    n3049 = local read "RUN"() -> (w4013:bool)
    n3050 = local read "Auto Start Temp"() -> (w4004:bool)
    n3051 = local read "Auto Start Test"() -> (w4012:bool)
    n3052 = local read "START TEMP"() -> (w4002:bool)
    n3053 = And(x=w4004, y=w4012) -> (x .and. y?=w4005:bool)
    n3054 = Or(x=w4013, y=w4005) -> (x .or. y?=w4014:bool)
    n3055 = And(x=w4014, y=w4002) -> (x .and. y?=w4001:bool)
    n3056 = And(x=w4003, y=w4002) -> (x .and. y?=w4000:bool)
    n3057 = Or(x=w4000, y=w4001) -> (x .or. y?=w3999:bool)
    n3058 = Wait (ms)(milliseconds to wait="milliseconds to wait") -> ()  [unwired: 1 out]
    n3059 = case shown="True" w3999 {
      tunnel: [400.0 ("out_vc_cmd") w4034] -> w4006
      tunnel: [w4018 w4036] -> w4007
      tunnel: [w4018 w4035] -> w4008
      tunnel: w4011 -> [_ w4025]
      tunnel: w4010 -> [_ w4024]
      tunnel: w4009 -> [_ w4023]
      tunnel: w4003 -> [_ w4019]
      frame False {
        w4018 = 0.0 ("error_out")
      }
      frame True {
        n3060 = case shown="True" w4019 {
          tunnel: [w4043 1.0] -> w4021
          frame False {
            n3061 = local read "Set Strk"() -> (w4042:dbl)
            n3062 = Add(x=w4042, y="Add up Stroke") -> (x+y=w4043:dbl)
          }
          frame True {
          }
        }
        n3063 = local read "LVDT STROKE"() -> (w4020:dbl)
        n3064 = formula code="// Zero-Hardcode Explicit Positional-Form PID Engine\n// Inputs: target_stroke, measured_stroke, dt, prev_error, integral_accumulator_in, prev_vc_cmd\n//         kp, ki, kd, max_step_change, max_amplitude, min_amplitude, startup_cmd\n// Outputs: vc_cmd, error_out, out_error, integral_accumulator_out, out_vc_cmd\n\n// 1. Calculate Tracking Error\nfloat current_error = target_stroke - measured_stroke;\nerror_out = current_error;\n\n// 2. Compute Proportional Term\nfloat p_term = kp * current_error;\n\n// 3. Compute Derivative Term\nfloat d_term = 0.0;\nif (dt > 0.0) {\n    d_term = kd * ((current_error - prev_error) / dt);\n}\n\n// 4. Update and Accumulate Integral Term\nfloat current_integral = integral_accumulator_in + (current_error * dt);\nfloat i_term = ki * current_integral;\n\n// 5. Calculate Ideal Target Command (Anchored by startup baseline)\nfloat ideal_command = startup_cmd + p_term + i_term + d_term;\n\n// 6. Apply Loop Rate Limiting FIRST \n// (Forces the command to climb gradually from prev_vc_cmd instead of jumping straight to max)\nfloat raw_adjustment = ideal_command - prev_vc_cmd;\n\nif (raw_adjustment > max_step_change) {\n    raw_adjustment = max_step_change;\n} else if (raw_adjustment < -max_step_change) {\n    raw_adjustment = -max_step_change;\n}\n\nfloat next_vc_cmd = prev_vc_cmd + raw_adjustment;\n\n// 7. Anti-Windup Protection & Final Output Safety Safeguard Clamping\n// (Back-calculating based on what we are ACTUALLY outputting)\nif (next_vc_cmd > max_amplitude) {\n    float excess = next_vc_cmd - max_amplitude;\n    if (ki > 0.0) {\n        current_integral -= excess / ki;\n    }\n    next_vc_cmd = max_amplitude;\n} else if (next_vc_cmd < min_amplitude) {\n    float excess = next_vc_cmd - min_amplitude;\n    if (ki > 0.0) {\n        current_integral -= excess / ki;\n    }\n    next_vc_cmd = min_amplitude;\n}\n\n// 8. Map to Shift Registers for memory persistence\nvc_cmd = next_vc_cmd;\nout_error = current_error;                   \nintegral_accumulator_out = current_integral;  \nout_vc_cmd = next_vc_cmd;"("target_stroke"=w4021, "measured_stroke"=w4020, "dt"="dt", "integral_accumulator_in"=w4024, "prev_error"=w4025, "prev_vc_cmd"=w4023, "kp"="kp", "ki"="ki", "kd"="kd", "max_step_change"="max_step_change", "max_amplitude"="max_amplitude", "min_amplitude"="min_amplitude", "startup_cmd"="startup_cmd") -> ("vc_cmd"=w4040:dbl, "out_error"=w4035:dbl, "integral_accumulator_out"=w4036:dbl, "out_vc_cmd"=w4034:dbl)  [unwired: 1 out]